vi "SaccadeAnalyser - Main.vi"(8 "error in (no error)":errorcluster, 11 "Data IN":T3={"Impulse Positions"=[{"Start"=5471, "End"=5813, "Impulse Plane"=enum."Yaw", "Impulse Direction +ve?"=FALSE, "Time offset"=0, "Amplitude offset"=0.0}, {"Start"=6974, "End"=7325, "Impulse Plane"=enum."Yaw", "Impulse Direction +ve?"=TRUE, "Time offset"=0, "Amplitude offset"=0.0}, {"Start"=7641, "End"=7980, "Impulse Plane"=enum."Yaw", "Impulse Direction +ve?"=FALSE, "Time offset"=0, "Amplitude offset"=0.0}, {"Start"=9060, "End"=9400, "Impulse Plane"=enum."Yaw", "Impulse Direction +ve?"=FALSE, "Time offset"=0, "Amplitude offset"=0.0}, {"Start"=9938, "End"=10282, "Impulse Plane"=enum."Yaw", "Impulse Direction +ve?"=FALSE, "Time offset"=0, "Amplitude offset"=0.0}, {"Start"=10800, "End"=11142, "Impulse Plane"=enum."Yaw", "Impulse Direction +ve?"=FALSE, "Time offset"=0, "Amplitude offset"=0.0}, {"Start"=11602, "End"=11942, "Impulse Plane"=enum."Yaw", "Impulse Direction +ve?"=TRUE, "Time offset"=0, "Amplitude offset"=0.0}, {"Start"=12449, "End"=12790, "Impulse Plane"=enum."Yaw", "Impulse Direction +ve?"=TRUE, "Time offset"=0, "Amplitude offset"=0.0}, {"Start"=13310, "End"=13653, "Impulse Plane"=enum."Yaw", "Impulse Direction +ve?"=TRUE, "Time offset"=0, "Amplitude offset"=0.0}, {"Start"=14191, "End"=14535, "Impulse Plane"=enum."Yaw", "Impulse Direction +ve?"=TRUE, "Time offset"=0, "Amplitude offset"=0.0}, {"Start"=15040, "End"=15380, "Impulse Plane"=enum."Yaw", "Impulse Direction +ve?"=FALSE, "Time offset"=0, "Amplitude offset"=0.0}, {"Start"=16780, "End"=17124, "Impulse Plane"=enum."Yaw", "Impulse Direction +ve?"=TRUE, "Time offset"=0, "Amplitude offset"=0.0}, {"Start"=17572, "End"=17913, "Impulse Plane"=enum."Yaw", "Impulse Direction +ve?"=FALSE, "Time offset"=0, "Amplitude offset"=0.0}, {"Start"=18369, "End"=18713, "Impulse Plane"=enum."Yaw", "Impulse Direction +ve?"=FALSE, "Time offset"=0, "Amplitude offset"=0.0}, {"Start"=19174, "End"=19519, "Impulse Plane"=enum."Yaw", "Impulse Direction +ve?"=FALSE, "Time offset"=0, "Amplitude offset"=0.0}, {"Start"=19928, "End"=20270, "Impulse Plane"=enum."Yaw", "Impulse Direction +ve?"=TRUE, "Time offset"=0, "Amplitude offset"=0.0}, {"Start"=20762, "End"=21121, "Impulse Plane"=enum."Yaw", "Impulse Direction +ve?"=FALSE, "Time offset"=0, "Amplitude offset"=0.0}, {"Start"=21554, "End"=21888, "Impulse Plane"=enum."Yaw", "Impulse Direction +ve?"=FALSE, "Time offset"=0, "Amplitude offset"=0.0}, {"Start"=22293, "End"=22639, "Impulse Plane"=enum."Yaw", "Impulse Direction +ve?"=TRUE, "Time offset"=0, "Amplitude offset"=0.0}, {"Start"=23109, "End"=23464, "Impulse Plane"=enum."Yaw", "Impulse Direction +ve?"=TRUE, "Time offset"=0, "Amplitude offset"=0.0}, {"Start"=23868, "End"=24215, "Impulse Plane"=enum."Yaw", "Impulse Direction +ve?"=TRUE, "Time offset"=0, "Amplitude offset"=0.0}, {"Start"=24643, "End"=24992, "Impulse Plane"=enum."Yaw", "Impulse Direction +ve?"=FALSE, "Time offset"=0, "Amplitude offset"=0.0}, {"Start"=25685, "End"=26023, "Impulse Plane"=enum."Yaw", "Impulse Direction +ve?"=FALSE, "Time offset"=0, "Amplitude offset"=0.0}, {"Start"=26431, "End"=26768, "Impulse Plane"=enum."Yaw", "Impulse Direction +ve?"=FALSE, "Time offset"=0, "Amplitude offset"=0.0}, {"Start"=27251, "End"=27595, "Impulse Plane"=enum."Yaw", "Impulse Direction +ve?"=FALSE, "Time offset"=0, "Amplitude offset"=0.0}, {"Start"=28832, "End"=29180, "Impulse Plane"=enum."Yaw", "Impulse Direction +ve?"=TRUE, "Time offset"=0, "Amplitude offset"=0.0}, {"Start"=31028, "End"=31383, "Impulse Plane"=enum."LARP", "Impulse Direction +ve?"=FALSE, "Time offset"=0, "Amplitude offset"=0.0}, {"Start"=32603, "End"=32936, "Impulse Plane"=enum."LARP", "Impulse Direction +ve?"=TRUE, "Time offset"=0, "Amplitude offset"=0.0}, {"Start"=33445, "End"=33779, "Impulse Plane"=enum."LARP", "Impulse Direction +ve?"=TRUE, "Time offset"=0, "Amplitude offset"=0.0}, {"Start"=34276, "End"=34629, "Impulse Plane"=enum."LARP", "Impulse Direction +ve?"=FALSE, "Time offset"=0, "Amplitude offset"=0.0}, {"Start"=35114, "End"=35460, "Impulse Plane"=enum."LARP", "Impulse Direction +ve?"=FALSE, "Time offset"=0, "Amplitude offset"=0.0}, {"Start"=35981, "End"=36324, "Impulse Plane"=enum."LARP", "Impulse Direction +ve?"=TRUE, "Time offset"=0, "Amplitude offset"=0.0}, {"Start"=36920, "End"=37249, "Impulse Plane"=enum."LARP", "Impulse Direction +ve?"=TRUE, "Time offset"=0, "Amplitude offset"=0.0}, {"Start"=37988, "End"=38322, "Impulse Plane"=enum."LARP", "Impulse Direction +ve?"=TRUE, "Time offset"=0, "Amplitude offset"=0.0}, {"Start"=38964, "End"=39324, "Impulse Plane"=enum."LARP", "Impulse Direction +ve?"=FALSE, "Time offset"=0, "Amplitude offset"=0.0}, {"Start"=39948, "End"=40284, "Impulse Plane"=enum."LARP", "Impulse Direction +ve?"=TRUE, "Time offset"=0, "Amplitude offset"=0.0}, {"Start"=40958, "End"=41293, "Impulse Plane"=enum."LARP", "Impulse Direction +ve?"=TRUE, "Time offset"=0, "Amplitude offset"=0.0}, {"Start"=41899, "End"=42229, "Impulse Plane"=enum."LARP", "Impulse Direction +ve?"=TRUE, "Time offset"=0, "Amplitude offset"=0.0}, {"Start"=42801, "End"=43154, "Impulse Plane"=enum."LARP", "Impulse Direction +ve?"=FALSE, "Time offset"=0, "Amplitude offset"=0.0}, {"Start"=43641, "End"=43980, "Impulse Plane"=enum."LARP", "Impulse Direction +ve?"=TRUE, "Time offset"=0, "Amplitude offset"=0.0}, {"Start"=44466, "End"=44821, "Impulse Plane"=enum."LARP", "Impulse Direction +ve?"=FALSE, "Time offset"=0, "Amplitude offset"=0.0}, {"Start"=45388, "End"=45722, "Impulse Plane"=enum."LARP", "Impulse Direction +ve?"=TRUE, "Time offset"=0, "Amplitude offset"=0.0}, {"Start"=46149, "End"=46510, "Impulse Plane"=enum."LARP", "Impulse Direction +ve?"=FALSE, "Time offset"=0, "Amplitude offset"=0.0}, {"Start"=47874, "End"=48206, "Impulse Plane"=enum."LARP", "Impulse Direction +ve?"=TRUE, "Time offset"=0, "Amplitude offset"=0.0}, {"Start"=50143, "End"=50479, "Impulse Plane"=enum."RALP", "Impulse Direction +ve?"=TRUE, "Time offset"=0, "Amplitude offset"=0.0}, {"Start"=50976, "End"=51310, "Impulse Plane"=enum."RALP", "Impulse Direction +ve?"=FALSE, "Time offset"=0, "Amplitude offset"=0.0}, {"Start"=51892, "End"=52226, "Impulse Plane"=enum."RALP", "Impulse Direction +ve?"=FALSE, "Time offset"=0, "Amplitude offset"=0.0}, {"Start"=52839, "End"=53171, "Impulse Plane"=enum."RALP", "Impulse Direction +ve?"=FALSE, "Time offset"=0, "Amplitude offset"=0.0}, {"Start"=53676, "End"=54012, "Impulse Plane"=enum."RALP", "Impulse Direction +ve?"=TRUE, "Time offset"=0, "Amplitude offset"=0.0}, {"Start"=54530, "End"=54877, "Impulse Plane"=enum."RALP", "Impulse Direction +ve?"=FALSE, "Time offset"=0, "Amplitude offset"=0.0}, {"Start"=55371, "End"=55711, "Impulse Plane"=enum."RALP", "Impulse Direction +ve?"=TRUE, "Time offset"=0, "Amplitude offset"=0.0}, {"Start"=56153, "End"=56482, "Impulse Plane"=enum."RALP", "Impulse Direction +ve?"=FALSE, "Time offset"=0, "Amplitude offset"=0.0}, {"Start"=57053, "End"=57390, "Impulse Plane"=enum."RALP", "Impulse Direction +ve?"=FALSE, "Time offset"=0, "Amplitude offset"=0.0}, {"Start"=57954, "End"=58292, "Impulse Plane"=enum."RALP", "Impulse Direction +ve?"=FALSE, "Time offset"=0, "Amplitude offset"=0.0}, {"Start"=58794, "End"=59130, "Impulse Plane"=enum."RALP", "Impulse Direction +ve?"=TRUE, "Time offset"=0, "Amplitude offset"=0.0}, {"Start"=59587, "End"=59931, "Impulse Plane"=enum."RALP", "Impulse Direction +ve?"=TRUE, "Time offset"=0, "Amplitude offset"=0.0}, {"Start"=60399, "End"=60744, "Impulse Plane"=enum."RALP", "Impulse Direction +ve?"=FALSE, "Time offset"=0, "Amplitude offset"=0.0}, {"Start"=61218, "End"=61559, "Impulse Plane"=enum."RALP", "Impulse Direction +ve?"=FALSE, "Time offset"=0, "Amplitude offset"=0.0}, {"Start"=62100, "End"=62442, "Impulse Plane"=enum."RALP", "Impulse Direction +ve?"=FALSE, "Time offset"=0, "Amplitude offset"=0.0}, {"Start"=62989, "End"=63322, "Impulse Plane"=enum."RALP", "Impulse Direction +ve?"=FALSE, "Time offset"=0, "Amplitude offset"=0.0}, {"Start"=63787, "End"=64136, "Impulse Plane"=enum."RALP", "Impulse Direction +ve?"=TRUE, "Time offset"=0, "Amplitude offset"=0.0}, {"Start"=64603, "End"=64953, "Impulse Plane"=enum."RALP", "Impulse Direction +ve?"=FALSE, "Time offset"=0, "Amplitude offset"=0.0}, {"Start"=65462, "End"=65795, "Impulse Plane"=enum."RALP", "Impulse Direction +ve?"=FALSE, "Time offset"=0, "Amplitude offset"=0.0}, {"Start"=66308, "End"=66645, "Impulse Plane"=enum."RALP", "Impulse Direction +ve?"=FALSE, "Time offset"=0, "Amplitude offset"=0.0}, {"Start"=67052, "End"=67402, "Impulse Plane"=enum."RALP", "Impulse Direction +ve?"=TRUE, "Time offset"=0, "Amplitude offset"=0.0}], "No. Imp"=15, "Parameter Time Series"=[{"time offset"=0.0, "Offset"=0.0, "Gain"=1.0, "inverse"=FALSE, "filter data"=FALSE, "dots"=FALSE, "interpolate"=FALSE, "List 1"=5, "Color Box"=6618880, "Boolean"=TRUE}, {"time offset"=0.0, "Offset"=0.0, "Gain"=1.0, "inverse"=FALSE, "filter data"=FALSE, "dots"=FALSE, "interpolate"=FALSE, "List 1"=6, "Color Box"=6618880, "Boolean"=FALSE}, {"time offset"=0.0, "Offset"=0.0, "Gain"=1.0, "inverse"=FALSE, "filter data"=FALSE, "dots"=FALSE, "interpolate"=FALSE, "List 1"=7, "Color Box"=6618880, "Boolean"=FALSE}, {"time offset"=0.0, "Offset"=0.0, "Gain"=1.0, "inverse"=FALSE, "filter data"=FALSE, "dots"=FALSE, "interpolate"=FALSE, "List 1"=13, "Color Box"=16777224, "Boolean"=TRUE}, {"time offset"=0.0, "Offset"=0.0, "Gain"=1.0, "inverse"=FALSE, "filter data"=FALSE, "dots"=FALSE, "interpolate"=FALSE, "List 1"=14, "Color Box"=16777224, "Boolean"=FALSE}, {"time offset"=0.0, "Offset"=0.0, "Gain"=1.0, "inverse"=FALSE, "filter data"=FALSE, "dots"=FALSE, "interpolate"=FALSE, "List 1"=15, "Color Box"=16777224, "Boolean"=FALSE}], "Parameter Impuls Series"=[{"Color"=6618880, "Visible"=TRUE, "Channel"=1, "Invert"=FALSE, "Desaccade"=FALSE, "Offset"=0.0, "Gain"=1.0}, {"Color"=6618880, "Visible"=FALSE, "Channel"=6, "Invert"=FALSE, "Desaccade"=FALSE, "Offset"=0.0, "Gain"=1.0}, {"Color"=6618880, "Visible"=FALSE, "Channel"=7, "Invert"=FALSE, "Desaccade"=FALSE, "Offset"=0.0, "Gain"=1.0}, {"Color"=16777224, "Visible"=TRUE, "Channel"=13, "Invert"=FALSE, "Desaccade"=FALSE, "Offset"=0.0, "Gain"=1.0}, {"Color"=16777224, "Visible"=FALSE, "Channel"=14, "Invert"=FALSE, "Desaccade"=FALSE, "Offset"=0.0, "Gain"=1.0}, {"Color"=16777224, "Visible"=FALSE, "Channel"=15, "Invert"=FALSE, "Desaccade"=FALSE, "Offset"=0.0, "Gain"=1.0}], "Experiment Parameters"={"Freq"=0.0, "Vel"=0, "Acc"=0, "Stimulus"="Head Impulse"}, "Autosort File"=refnum, "Data File"={"Data Channels"=array34x71049[2415666 elements], "Sample Rate"=500, "Channel List"=["Hz Position-in-Head", "Hz Velocity-in-Head", "Hy Position-in-Head", "Hy Velocity-in-Head", "Hx Position-in-Head", "Hx Velocity-in-Head", "Hl Velocity-in-Head", "Hr Velocity-in-Head", "Lx Position-in-Head", "Ly Position-in-Head", "Lz Position-in-Head", "Lx Velocity-in-Head", "Ly Velocity-in-Head", "Lz Velocity-in-Head", "Ll Velocity-in-Head", "Lr Velocity-in-Head", "Rx Position-in-Head", "Ry Position-in-Head", "Rz Position-in-Head", "Rx Velocity-in-Head", "Ry Velocity-in-Head", "Rz Velocity-in-Head", "Rl Velocity-in-Head", "Rr Velocity-in-Head", "Target on/off", "aux input 1", "aux input 2", " ", "", "", "", "Target Hor", "Target Ver", ""]}, "Experiment data path"=path "C:/Users/w.figtree/Desktop/Coils Data/3", "Image data path"=path "/Macintosh HD/Users/patrick/Studium/Diploma Thesis/Data Analysis", "LVS data path"=path "/Macintosh HD/Users/patrick/Studium/Diploma Thesis/Data Analysis", "Raw copy path"=path "/Macintosh HD/Users/patrick/Studium/Diploma Thesis/Data Analysis", "filename"="passive_lvs.lvs", "desaccading parameters"={"Tolerance"=3, "Acc Range"=7000.0, "Sample Rate"=500, "Impulse Plane 2"=enum."Yaw", "Impulse dir"=FALSE}, "Experiment Parameters 2"={"Subject"="SE Trial Short Term", "Strain"="", "Rotation plane"="", "Experimenter"=" ", "Trial"=0.0, "Time"=0.0}, "Excel"={"Excel._Application"=refnum, "Use Excel"=TRUE, "Worksheet SINE"=refnum, "Row SINE"=0, "Worksheet TRANS"=refnum, "Row TRANS"=0}, "Session Config File"=refnum, "Autosort Parameter Set"=4, "EMA Version"="EMA 2016a", "desacc "={"Threshold 1 [Acc]"=7000.0, "Threshold 2 [% of TH1]"=60, "tolerance"=3, "Search WD "=0.1, " always use TH2"=FALSE, "Range"=3.0, "Max time"=120.0, "Min time"=20.0, "Velocity Threshold"=150}, "Cycle Nr for Saccades"={"POS"=0, "NEG"=0}, "calibration name"="u_calibration_1_p00001s001_calib.mat", "Excel"=refnum} {"Parameter Time Series"."time offset" format="%.3f"; "Parameter Time Series"."Gain" format="%.1f"; "Parameter Time Series"."Offset" format="%.1f"; "Parameter Time Series"."List 1" items=["Motor-Pos", "Motor-Vel", "Lx Position-in-Head", "Ly Position-in-Head", "Lz Position-in-Head", "Lx Velocity-in-Head", "Ly Velocity-in-Head", "Lz Velocity-in-Head", "Ll Velocity-in-Head", "Lr Velocity-in-Head", "Lx Accel-in-Head", "Ly Accel-in-Head", "Lz Accel-in-Head", "Rx Position-in-Head", "Ry Position-in-Head", "Rz Position-in-Head", "Rx Velocity-in-Head", "Ry Velocity-in-Head", "Rz Velocity-in-Head", "Rl Velocity-in-Head", "Rr Velocity-in-Head", "Rx Accel-in-Head", "Ry Accel-in-Head", "Rz Accel-in-Head", "Global Trigger", "", "", ""]; "Parameter Impuls Series"."Gain" format="%.1f"; "Parameter Impuls Series"."Offset" format="%.1f"}) -> (0 "error out":errorcluster, 3 "Data OUT":T3={"Impulse Positions"=[{"Start"=5471, "End"=5813, "Impulse Plane"=enum."Yaw", "Impulse Direction +ve?"=FALSE, "Time offset"=0, "Amplitude offset"=0.0}, {"Start"=6974, "End"=7325, "Impulse Plane"=enum."Yaw", "Impulse Direction +ve?"=TRUE, "Time offset"=0, "Amplitude offset"=0.0}, {"Start"=7641, "End"=7980, "Impulse Plane"=enum."Yaw", "Impulse Direction +ve?"=FALSE, "Time offset"=0, "Amplitude offset"=0.0}, {"Start"=9060, "End"=9400, "Impulse Plane"=enum."Yaw", "Impulse Direction +ve?"=FALSE, "Time offset"=0, "Amplitude offset"=0.0}, {"Start"=9938, "End"=10282, "Impulse Plane"=enum."Yaw", "Impulse Direction +ve?"=FALSE, "Time offset"=0, "Amplitude offset"=0.0}, {"Start"=10800, "End"=11142, "Impulse Plane"=enum."Yaw", "Impulse Direction +ve?"=FALSE, "Time offset"=0, "Amplitude offset"=0.0}, {"Start"=11602, "End"=11942, "Impulse Plane"=enum."Yaw", "Impulse Direction +ve?"=TRUE, "Time offset"=0, "Amplitude offset"=0.0}, {"Start"=12449, "End"=12790, "Impulse Plane"=enum."Yaw", "Impulse Direction +ve?"=TRUE, "Time offset"=0, "Amplitude offset"=0.0}, {"Start"=13310, "End"=13653, "Impulse Plane"=enum."Yaw", "Impulse Direction +ve?"=TRUE, "Time offset"=0, "Amplitude offset"=0.0}, {"Start"=14191, "End"=14535, "Impulse Plane"=enum."Yaw", "Impulse Direction +ve?"=TRUE, "Time offset"=0, "Amplitude offset"=0.0}, {"Start"=15040, "End"=15380, "Impulse Plane"=enum."Yaw", "Impulse Direction +ve?"=FALSE, "Time offset"=0, "Amplitude offset"=0.0}, {"Start"=16780, "End"=17124, "Impulse Plane"=enum."Yaw", "Impulse Direction +ve?"=TRUE, "Time offset"=0, "Amplitude offset"=0.0}, {"Start"=17572, "End"=17913, "Impulse Plane"=enum."Yaw", "Impulse Direction +ve?"=FALSE, "Time offset"=0, "Amplitude offset"=0.0}, {"Start"=18369, "End"=18713, "Impulse Plane"=enum."Yaw", "Impulse Direction +ve?"=FALSE, "Time offset"=0, "Amplitude offset"=0.0}, {"Start"=19174, "End"=19519, "Impulse Plane"=enum."Yaw", "Impulse Direction +ve?"=FALSE, "Time offset"=0, "Amplitude offset"=0.0}, {"Start"=19928, "End"=20270, "Impulse Plane"=enum."Yaw", "Impulse Direction +ve?"=TRUE, "Time offset"=0, "Amplitude offset"=0.0}, {"Start"=20762, "End"=21121, "Impulse Plane"=enum."Yaw", "Impulse Direction +ve?"=FALSE, "Time offset"=0, "Amplitude offset"=0.0}, {"Start"=21554, "End"=21888, "Impulse Plane"=enum."Yaw", "Impulse Direction +ve?"=FALSE, "Time offset"=0, "Amplitude offset"=0.0}, {"Start"=22293, "End"=22639, "Impulse Plane"=enum."Yaw", "Impulse Direction +ve?"=TRUE, "Time offset"=0, "Amplitude offset"=0.0}, {"Start"=23109, "End"=23464, "Impulse Plane"=enum."Yaw", "Impulse Direction +ve?"=TRUE, "Time offset"=0, "Amplitude offset"=0.0}, {"Start"=23868, "End"=24215, "Impulse Plane"=enum."Yaw", "Impulse Direction +ve?"=TRUE, "Time offset"=0, "Amplitude offset"=0.0}, {"Start"=24643, "End"=24992, "Impulse Plane"=enum."Yaw", "Impulse Direction +ve?"=FALSE, "Time offset"=0, "Amplitude offset"=0.0}, {"Start"=25685, "End"=26023, "Impulse Plane"=enum."Yaw", "Impulse Direction +ve?"=FALSE, "Time offset"=0, "Amplitude offset"=0.0}, {"Start"=26431, "End"=26768, "Impulse Plane"=enum."Yaw", "Impulse Direction +ve?"=FALSE, "Time offset"=0, "Amplitude offset"=0.0}, {"Start"=27251, "End"=27595, "Impulse Plane"=enum."Yaw", "Impulse Direction +ve?"=FALSE, "Time offset"=0, "Amplitude offset"=0.0}, {"Start"=28832, "End"=29180, "Impulse Plane"=enum."Yaw", "Impulse Direction +ve?"=TRUE, "Time offset"=0, "Amplitude offset"=0.0}, {"Start"=31028, "End"=31383, "Impulse Plane"=enum."LARP", "Impulse Direction +ve?"=FALSE, "Time offset"=0, "Amplitude offset"=0.0}, {"Start"=32603, "End"=32936, "Impulse Plane"=enum."LARP", "Impulse Direction +ve?"=TRUE, "Time offset"=0, "Amplitude offset"=0.0}, {"Start"=33445, "End"=33779, "Impulse Plane"=enum."LARP", "Impulse Direction +ve?"=TRUE, "Time offset"=0, "Amplitude offset"=0.0}, {"Start"=34276, "End"=34629, "Impulse Plane"=enum."LARP", "Impulse Direction +ve?"=FALSE, "Time offset"=0, "Amplitude offset"=0.0}, {"Start"=35114, "End"=35460, "Impulse Plane"=enum."LARP", "Impulse Direction +ve?"=FALSE, "Time offset"=0, "Amplitude offset"=0.0}, {"Start"=35981, "End"=36324, "Impulse Plane"=enum."LARP", "Impulse Direction +ve?"=TRUE, "Time offset"=0, "Amplitude offset"=0.0}, {"Start"=36920, "End"=37249, "Impulse Plane"=enum."LARP", "Impulse Direction +ve?"=TRUE, "Time offset"=0, "Amplitude offset"=0.0}, {"Start"=37988, "End"=38322, "Impulse Plane"=enum."LARP", "Impulse Direction +ve?"=TRUE, "Time offset"=0, "Amplitude offset"=0.0}, {"Start"=38964, "End"=39324, "Impulse Plane"=enum."LARP", "Impulse Direction +ve?"=FALSE, "Time offset"=0, "Amplitude offset"=0.0}, {"Start"=39948, "End"=40284, "Impulse Plane"=enum."LARP", "Impulse Direction +ve?"=TRUE, "Time offset"=0, "Amplitude offset"=0.0}, {"Start"=40958, "End"=41293, "Impulse Plane"=enum."LARP", "Impulse Direction +ve?"=TRUE, "Time offset"=0, "Amplitude offset"=0.0}, {"Start"=41899, "End"=42229, "Impulse Plane"=enum."LARP", "Impulse Direction +ve?"=TRUE, "Time offset"=0, "Amplitude offset"=0.0}, {"Start"=42801, "End"=43154, "Impulse Plane"=enum."LARP", "Impulse Direction +ve?"=FALSE, "Time offset"=0, "Amplitude offset"=0.0}, {"Start"=43641, "End"=43980, "Impulse Plane"=enum."LARP", "Impulse Direction +ve?"=TRUE, "Time offset"=0, "Amplitude offset"=0.0}, {"Start"=44466, "End"=44821, "Impulse Plane"=enum."LARP", "Impulse Direction +ve?"=FALSE, "Time offset"=0, "Amplitude offset"=0.0}, {"Start"=45388, "End"=45722, "Impulse Plane"=enum."LARP", "Impulse Direction +ve?"=TRUE, "Time offset"=0, "Amplitude offset"=0.0}, {"Start"=46149, "End"=46510, "Impulse Plane"=enum."LARP", "Impulse Direction +ve?"=FALSE, "Time offset"=0, "Amplitude offset"=0.0}, {"Start"=47874, "End"=48206, "Impulse Plane"=enum."LARP", "Impulse Direction +ve?"=TRUE, "Time offset"=0, "Amplitude offset"=0.0}, {"Start"=50143, "End"=50479, "Impulse Plane"=enum."RALP", "Impulse Direction +ve?"=TRUE, "Time offset"=0, "Amplitude offset"=0.0}, {"Start"=50976, "End"=51310, "Impulse Plane"=enum."RALP", "Impulse Direction +ve?"=FALSE, "Time offset"=0, "Amplitude offset"=0.0}, {"Start"=51892, "End"=52226, "Impulse Plane"=enum."RALP", "Impulse Direction +ve?"=FALSE, "Time offset"=0, "Amplitude offset"=0.0}, {"Start"=52839, "End"=53171, "Impulse Plane"=enum."RALP", "Impulse Direction +ve?"=FALSE, "Time offset"=0, "Amplitude offset"=0.0}, {"Start"=53676, "End"=54012, "Impulse Plane"=enum."RALP", "Impulse Direction +ve?"=TRUE, "Time offset"=0, "Amplitude offset"=0.0}, {"Start"=54530, "End"=54877, "Impulse Plane"=enum."RALP", "Impulse Direction +ve?"=FALSE, "Time offset"=0, "Amplitude offset"=0.0}, {"Start"=55371, "End"=55711, "Impulse Plane"=enum."RALP", "Impulse Direction +ve?"=TRUE, "Time offset"=0, "Amplitude offset"=0.0}, {"Start" (continued)
69.17902917715358, 60.07870769971235, 48.3314198066639, 35.33337743696967, 22.457297716500758, 10.830764991263301, 1.2205986166028433, -6.0146150669211735, -10.892007595538576, -13.694807591178186, -14.851804332650717]}, {[528.0, 530.0, 532.0, 534.0, 536.0, 538.0, 540.0, 542.0, 544.0, 546.0, 548.0, 550.0, 552.0, 554.0, 556.0, 558.0, 560.0, 562.0, 564.0, 566.0000000000001, 568.0000000000001, 570.0000000000001, 572.0000000000001, 574.0000000000001, 576.0000000000001], [-9.527579454864409, -10.577125665129762, -11.131145103375022, -10.584223908245097, -8.348654243177833, -4.004783979283369, 2.5647973786029565, 11.078531818240757, 20.82241073585996, 30.726895783053166, 39.52405801175928, 45.95532417764138, 49.01661960104225, 48.16011299362397, 43.404321671726706, 35.33378791984829, 25.00271709876472, 13.751187200019555, 2.9552038725955043, -6.2063612167617315, -12.921399963820624, -16.839745644954295, -18.071940127929174, -17.104117050659703, -14.654065025286862]}, {[582.0, 584.0, 586.0, 588.0, 590.0, 592.0, 594.0, 596.0, 598.0, 600.0, 602.0, 604.0, 606.0, 608.0, 610.0, 612.0, 614.0, 616.0, 618.0, 620.0, 622.0, 624.0, 626.0, 628.0, 630.0, 632.0, 634.0], [-1.6706932697042873, -3.3455075811287243, -4.473678994481653, -4.396585575335241, -2.4684369191577247, 1.8007580481050427, 8.594949141623625, 17.683034583489096, 28.386913259392607, 39.64175106168615, 50.1408646696851, 58.542587224043245, 63.692457661993835, 64.82578843596133, 61.715514730847474, 54.70461631035364, 44.63458910283943, 32.701219003695016, 20.241708562239864, 8.517446480794685, -1.459609986588287, -9.042719586196379, -13.99397311102634, -16.457101162835592, -16.860363274420028, -15.79407496046417, -13.893778016469078]}, {[474.00000000000006, 476.00000000000006, 478.00000000000006, 480.00000000000006, 482.00000000000006, 484.00000000000006, 486.00000000000006, 488.00000000000006, 490.00000000000006, 492.00000000000006, 494.00000000000006, 496.00000000000006, 498.00000000000006, 500.0, 502.0, 504.0, 506.0, 508.0, 510.0, 512.0, 514.0, 516.0, 518.0, 520.0, 522.0, 524.0, 526.0], [-5.437581721706813, -7.532853000022355, -9.084142746911153, -9.250990048241723, -7.178612795093302, -2.1928649146719312, 6.0140070464960305, 17.233642801887164, 30.675418822257488, 45.01795262576213, 58.59539464359083, 69.67881969840226, 76.76808432526585, 78.8729582975258, 75.70844363988871, 67.73827863726395, 56.07362169336059, 42.251256479738785, 27.958663515334496, 14.743425419148696, 3.764146667680771, -4.34286902425044, -9.463854697830513, -11.922815948161967, -12.338815179197, -11.433286382606058, -9.865105428418754]}, {[564.0, 566.0000000000001, 568.0000000000001, 570.0000000000001, 572.0000000000001, 574.0000000000001, 576.0000000000001, 578.0000000000001, 580.0000000000001, 582.0000000000001, 584.0000000000001, 586.0000000000001, 588.0000000000001, 590.0000000000001, 592.0000000000001, 594.0000000000001, 596.0000000000001, 598.0000000000001, 600.0000000000001, 602.0000000000001, 604.0000000000001, 606.0000000000001, 608.0000000000001, 610.0000000000001, 612.0000000000001, 614.0000000000001, 616.0000000000001], [-9.080046765081676, -10.678128490411645, -11.6707704891704, -11.469856027373027, -9.5158355327974, -5.413075001297588, 0.9434399127670785, 9.27089343229068, 18.885806355145963, 28.78298155221996, 37.772096486182164, 44.65829905955033, 48.46266031046852, 48.61309811323283, 45.03993832436139, 38.180486368387854, 28.912453408573064, 18.402759339239452, 7.886075499642308, -1.5232402772824392, -8.985318767842745, -14.04591575558494, -16.647938966841256, -17.078934812254147, -15.873611988630202, -13.67825841551836, -11.126693516226487]}, {[518.0, 520.0, 522.0, 524.0, 526.0, 528.0, 530.0, 532.0, 534.0, 536.0, 538.0, 540.0, 542.0, 544.0, 546.0, 548.0, 550.0, 552.0, 554.0, 556.0, 558.0, 560.0, 562.0, 564.0, 566.0000000000001, 568.0000000000001, 570.0000000000001], [-11.4476193776905, -13.068851678881895, -13.862730914838576, -12.99963998702583, -9.694639981902103, -3.402083180014002, 6.032556885524558, 18.251678113366445, 32.3514578152284, 46.96196273804698, 60.41458212174757, 71.01485846520777, 77.33772940656948, 78.468047531521, 74.18538908447246, 65.01631412660365, 52.128564083566516, 37.14123702954777, 21.855399138477154, 7.934316510732438, -3.3578249787371295, -11.309186108976784, -15.805578117508423, -17.26506975033719, -16.46631522978143, -14.335344694369246, -11.750138041033814]}, {[498.0, 500.0, 502.0, 504.0, 506.0, 508.0, 510.0, 512.0, 514.0, 516.0, 518.0, 520.0, 522.0, 524.0, 526.0, 528.0, 530.0, 532.0, 534.0, 536.0, 538.0, 540.0, 542.0, 544.0, 546.0, 548.0, 550.0], [-0.012091313230288447, -1.7421638804518995, -3.0389623640143157, -3.245396673757427, -1.6948480326152768, 2.1384328191819306, 8.469521915823595, 17.087054841087145, 27.315418397717107, 38.05757322742741, 47.94620610349132, 55.57948276025742, 59.777197966332054, 59.80311209652382, 55.50908234625477, 47.38023657915541, 36.450375305358186, 24.101455072542254, 11.809603266892601, 0.8926245665691606, -7.699270570892281, -13.502462377823814, -16.541721280039642, -17.24392262332151, -16.284433481949875, -14.412508844326226, -12.2971280291156]}, {[554.0, 556.0, 558.0, 560.0, 562.0, 564.0, 566.0000000000001, 568.0000000000001, 570.0000000000001, 572.0000000000001, 574.0000000000001, 576.0000000000001, 578.0000000000001, 580.0000000000001, 582.0000000000001, 584.0000000000001, 586.0000000000001, 588.0000000000001, 590.0000000000001, 592.0000000000001, 594.0000000000001, 596.0000000000001, 598.0000000000001, 600.0000000000001, 602.0000000000001, 604.0000000000001, 606.0000000000001], [-4.522231629389672, -6.099356541635326, -7.033837566184765, -6.530522920748879, -3.7817473387038465, 1.850754719532537, 10.642426983685915, 22.365587411552568, 36.23501199222388, 50.94709617216887, 64.84101602206391, 76.17471628829185, 83.41922636843152, 85.51991298092757, 82.09980450239388, 73.53608919952723, 60.89872991717725, 45.758420318077484, 29.907265361805152, 15.058407133564199, 2.5737382904767507, -6.715899336652479, -12.57598159697483, -15.3246447501556, -15.686631915632411, -14.574916517929267, -12.872113276125042]}, {[520.0, 522.0, 524.0, 526.0, 528.0, 530.0, 532.0, 534.0, 536.0, 538.0, 540.0, 542.0, 544.0, 546.0, 548.0, 550.0, 552.0, 554.0, 556.0, 558.0, 560.0, 562.0, 564.0, 566.0000000000001, 568.0000000000001, 570.0000000000001, 572.0000000000001], [-7.500446204332798, -8.149769047301705, -8.599376666418916, -8.441802829436932, -7.230678641797557, -4.591111049576478, -0.3257926505220681, 5.492766404293648, 12.473385539202374, 19.915354566494162, 26.90003759789026, 32.44825466462659, 35.686366632079164, 36.01778064482943, 33.26105823585337, 27.682301361140524, 19.94926639447815, 11.04003883936146, 2.0609526551163264, -5.955707230259444, -12.201977016180082, -16.200494428585834, -17.8432974158248, -17.366919156986576, -15.269937620203358, -12.180213398484451, -8.726924390155432]}, {[552.0, 554.0, 556.0, 558.0, 560.0, 562.0, 564.0, 566.0000000000001, 568.0000000000001, 570.0000000000001, 572.0000000000001, 574.0000000000001, 576.0000000000001, 578.0000000000001, 580.0000000000001, 582.0000000000001, 584.0000000000001, 586.0000000000001, 588.0000000000001, 590.0000000000001, 592.0000000000001, 594.0000000000001, 596.0000000000001, 598.0000000000001, 600.0000000000001, 602.0000000000001, 604.0000000000001], [-7.176035360345667, -7.398600739376963, -7.3767525082011804, -6.7782328355304795, -5.314655641339901, -2.8256467063059447, 0.6726090248953283, 4.98148672460113, 9.750320796626117, 14.530187559033408, 18.84255920678958, 22.26067541171979, 24.468305768199688, 25.29294718130975, 24.725614427990152, 22.9030335665933, 20.082655608922238, 16.606151876437476, 12.82963888753322, 9.079726996951507, 5.622531347536689, 2.6217090367480265, 0.13171202491932155, -1.8838458215461478, -3.5233802618856194, -4.91150074028557, -6.173130009585858]}, {[552.0, 554.0, 556.0, 558.0, 560.0, 562.0, 564.0, 566.0000000000001, 568.0000000000001, 570.0000000000001, 572.0000000000001, 574.0000000000001, 576.0000000000001, 578.0000000000001, 580.0000000000001, 582.0000000000001, 584.0000000000001, 586.0000000000001, 588.0000000000001, 590.0000000000001, 592.0000000000001, 594.0000000000001, 596.0000000000001, 598.0000000000001, 600.0000000000001, 602.0000000000001], [-7.038075410780015, -8.577769843416434, -9.850303709444205, -10.436079719799327, -9.89643731331821, -7.860113468983564, -4.139867507193869, 1.1836393543016275, 7.714366955283603, 14.747407872743832, 21.37706522917261, 26.656315254909103, 29.755925905755753, 30.1306788554151, 27.65294175194612, 22.631211021641793, 15.742249750023644, 7.917552080655157, 0.16434731585808038, -6.624286177975039, -11.814424012090928, -15.105823184589445, -16.53122154971252, -16.40521618929207, -15.215912519074433, -13.498067256588318]}, {[0.0, 2.0, 4.0, 6.0, 8.0, 10.0, 12.0, 14.0, 16.0, 18.000000000000004, 20.0, 22.0, 24.0, 26.000000000000004, 28.0, 30.0, 32.0, 34.0, 36.00000000000001, 38.0, 40.0, 42.0, 44.0, 46.0, 48.0, 50.0, 52.00000000000001, 54.0, 56.0, 58.0, 60.0, 62.0, 64.0, 66.0, 68.0, 70.0, 72.00000000000001, 74.0, 76.0, 78.0, 80.0, 82.0, 84.0, 86.0, 88.0, 90.0, 92.0, 94.0, 96.0, 98.0, 100.0, 102.00000000000001, 104.00000000000001, 106.0, 108.0, 110.0, 112.0, 114.0, 116.0, 118.00000000000001, 120.0, 122.0, 124.0, 126.0, 128.0, 130.0, 132.0, 134.0, 136.0, 138.0, 140.0, 142.00000000000003, 144.00000000000003, 146.0, 148.0, 150.0, 152.0, 154.0, 156.0, 158.0, 160.0, 162.0, 164.0, 166.0, 168.0, 170.0, 172.0, 174.00000000000003, 176.0, 178.0, 180.0, 182.0, 184.0, 186.0, 188.0, 190.0, 192.0, 194.0, 196.0, 198.0, 200.0, 202.0, 204.00000000000003, 206.00000000000003, 208.00000000000003, 210.0, 212.0, 214.0, 216.0, 218.0, 220.0, 222.0, 224.0, 226.0, 228.0, 230.0, 232.0, 234.0, 236.00000000000003, 238.00000000000003, 240.0, 242.0, 244.0, 246.0, 248.0, 250.0, 252.0, 254.0, 256.0, 258.0, 260.0, 262.0, 264.0, 266.0, 268.0, 270.0, 272.0, 274.0, 276.0, 278.0, 280.0, 282.0, 284.00000000000006, 286.00000000000006, 288.00000000000006, 290.0, 292.0, 294.0, 296.0, 298.0, 300.0, 302.0, 304.0, 306.0, 308.0, 310.0, 312.0, 314.0, 316.0, 318.0, 320.0, 322.0, 324.0, 326.0, 328.0, 330.0, 332.0, 334.0, 336.0, 338.0, 340.0, 342.0, 344.0, 346.00000000000006, 348.00000000000006, 350.00000000000006, 352.0, 354.0, 356.0, 358.0, 360.0, 362.0, 364.0, 366.0, 368.0, 370.0, 372.0, 374.0, 376.0, 378.0, 380.0, 382.0, 384.0, 386.0, 388.0, 390.0, 392.0, 394.0, 396.0, 398.0, 400.0, 402.0, 404.0, 406.0, 408.00000000000006, 410.00000000000006, 412.00000000000006, 414.00000000000006, 416.00000000000006, 418.0, 420.0, 422.0, 424.0, 426.0, 428.0, 430.0, 432.0, 434.0, 436.0, 438.0, 440.0, 442.0, 444.0, 446.0, 448.0, 450.0, 452.0, 454.0, 456.0, 458.0, 460.0, 462.0, 464.0, 466.0, 468.0, 470.00000000000006, 472.00000000000006, 474.00000000000006, 476.00000000000006, 478.00000000000006, 480.0, 482.0, 484.0, 486.0, 488.0, 490.0, 492.0, 494.0, 496.0, 498.0, 500.0, 502.0, 504.0, 506.0, 508.0, 510.0, 512.0, 514.0, 516.0, 518.0, 520.0, 522.0, 524.0, 526.0, 528.0, 530.0, 532.0, 534.0, 536.0, 538.0, 540.0, 542.0, 544.0, 546.0, 548.0, 550.0, 552.0, 554.0, 556.0, 558.0, 560.0, 562.0, 564.0, 566.0000000000001, 568.0000000000001, 570.0000000000001, 572.0000000000001, 574.0000000000001, 576.0000000000001, 578.0, 580.0, 582.0, 584.0, 586.0, 588.0, 590.0, 592.0, 594.0, 596.0, 598.0, 600.0, 602.0, 604.0, 606.0, 608.0, 610.0, 612.0, 614.0, 616.0, 618.0, 620.0, 622.0, 624.0, 626.0, 628.0, 630.0, 632.0, 634.0, 636.0, 638.0, 640.0, 642.0, 644.0, 646.0, 648.0, 650.0, 652.0, 654.0, 656.0, 658.0, 660.0, 662.0, 664.0, 666.0, 668.0], [-0.06389984985435682, -0.12570215489812853, -0.18723624777264014, -0.23828621839494524, -0.2694747074102395, -0.27642488116316066, -0.2565836311633518, -0.20727945016965776, -0.1343952403934754, -0.05130262808294894, 0.026136502806187067, 0.09013326590404347, 0.13607030565691858, 0.1528909675810457, 0.13442869149282366, 0.07988100427413869, -0.002401488036655408, -0.1022500676685194, -0.21797896262421368, -0.3388258429025601, -0.44434173621161754, -0.5193440654063686, -0.5441483456323404, -0.49032714150705736, -0.33793533239258977, -0.0807577811775344, 0.2709286369262154, 0.6842131468323549, 1.1059532487254442, 1.4712547669651963, 1.7184375078906475, 1.8037877183406046, 1.7165562417297897, 1.4906890339021412, 1.1962647788928518, 0.9219480164005205, 0.7556012152472324, 0.7566134320243072, 0.9375918220718509, 1.2604732475075489, 1.6373372725704858, 1.9502489127578508, 2.0859920093783213, 1.9667398372264877, 1.571410782977047, 0.9479237512795624, 0.20652338004889703, -0.5061423952844164, -1.036944621211461, -1.2653053318499596, -1.1309933377401444, -0.6366869285332228, 0.15166053693547, 1.1156729380654244, 2.11318603669417, 3.0055200477133646, 3.6859144692725643, 4.094720432450903, 4.215302256662561, 4.0766289401086775, 3.742633925618021, 3.30620501255844, 2.881439696264434, 2.574878674689037, 2.4803761037274317, 2.6706236208689536, 3.18368074995124, 4.007194511359277, 5.0710977588308666, 6.268854508144667, 7.469526323813759, 8.530376261036054, 9.342553263713715, 9.863799207277001, 10.123466542701575, 10.229880290219269, 10.354131182709867, 10.696877627531286, 11.45321245373188, 12.780097146857049, 14.755224840526338, 17.357696457903977, 20.48998681579132, 23.99995799476212, 27.706546163615634, 31.431952854451144, 35.04133998301175, 38.468242825404246, 41.71242171435395, 44.83963375223422, 47.96908344679959, 51.24060422237642, 54.79190574811583, 58.740443124718546, 63.155006680308226, 68.04465837590038, 73.3615702443747, 79.00358082817246, 84.83319830639687, 90.69733687089266, 96.4423992300049, 101.9432307418265, 107.12399871295318, 111.95524640951494, 116.44863508113531, 120.6472053453836, 124.60196091677193, 128.349142018269, 131.89713260435985, 135.21463691584137, 138.22863339329965, 140.84690778164585, 142.9860874893099, 144.58344412978295, 145.60554802558585, 146.06292399523926, 146.0050494698197, 145.49918498468293, 144.61919601487403, 143.4294723740994, 141.9684488682583, 140.25116736087017, 138.28057416903903, 136.05354532550473, 133.57377096057576, 130.8644435484759, 127.96387751830784, 124.91429647774994, 121.74804633491232, 118.48705031725001, 115.12902939470527, 111.63761756623985, 107.9664649494672, 104.08208868515223, 99.97245653901649, 95.64179125464611, 91.12366744477903, 86.48787454792571, 81.81316742172847, 77.17316323413405, 72.6261348434492, 68.19300745085101, 63.864589153901576, 59.612788560229006, 55.389694447532946, 51.14642940264445, 46.84700990973632, 42.46941103237013, 38.014749206524115, 33.516721174253604, 29.028002933027782, 24.607030786188567, 20.326059759819604, 16.26756107893855, 12.503978941178676, 9.094780849860012, 6.086096366431338, 3.49866889030888, 1.3247104029809376, -0.48371886388815666, -2.0177722903845234, -3.393651881805288, -4.733521672382471, -6.143625357696668, -7.698555384136507, -9.425089192371736, -11.291206743853799, -13.206870439337532, -15.03853142345734, -16.649724144701665, -17.932941410231564, -18.814981304641147, -19.281357424128956, -19.393016423724085, -19.26490623139781, -19.03918123787503, -18.857271067575972, -18.83815084441698, -19.048711735356235, -19.481946575012877, -20.070198718358654, -20.70829324652221, -21.278554039911622, -21.67428152886609, -21.82600379548085, -21.732919189201056, -21.45993044115803, -21.109104979904828, -20.78788405459494, -20.581721175833167, -20.54113979532611, -20.660261440958287, -20.86262045188685, -21.02819124115802, -21.03757725352456, -20.797510556960738, -20.26030784475326, -19.439735515361683, -18.408533466274093, -17.27478134191867, -16.154037997324632, -15.148545262331227, -14.31686352558911, -13.66225116467085, -13.15704653269165, -12.75387164805027, -12.392129406286909, -12.024811564114465, -11.63692544379666, -11.241171953338721, -10.863122731837592, -10.52960912628934, -10.258073831383156, -10.04868665772845, -9.879755866486377, -9.715367173222496, -9.52530000995492, -9.286537202165821, -8.984146165670936, -8.630912304170035, -8.267568565427151, -7.9366125762916955, -7.679960446571975, -7.542205570373248, -7.547693321484007, -7.684364581657373, -7.911633348135986, -8.179315069141527, -8.41855546194656, -8.549571489449557, -8.518307893037509, -8.302060451762626, -7.918675856486931, -7.436473975500149, -6.955523665965402, -6.58891068598745, -6.4467335298213095, -6.60563125019346, -7.073137408571714, -7.788658924187796, -8.634927391988677, -9.449305857255634, -10.061179740092758, -10.323049141832405, -10.146512866779464, -9.536370639676214, -8.592198325897762, -7.495574612435697, -6.498709060387066, -5.888672615388614, -5.9297582067843715, -6.801976189574921, -8.523709941509901, -10.902101120878495, -13.515153937729416, -15.705975171447783, -16.647195116153465, -15.47020228179682, -11.434549595782723, -4.102893640842959, 6.514226198648548, 19.860845176201657, 34.84648813171131, 49.95971640001052, 63.47724286885524, 73.74340864036043, 79.44374271664638, 79.83243426595925, 74.86210287260596, 65.19120077463768, 52.06529031428731, 37.08937138080604, 21.955981839601936, 8.17411492228468, -3.1425345306333585, -11.379811752888802, -16.44083754969223, -18.678736575190545, -18.73357784286452, -17.361621097688346, -15.295562056242597, -13.126955560682532, -11.25919027367259, -9.902590375807705, -9.105508127115133, -8.811095023693332, -8.908120326942106, -9.278464792543527, -9.809734471536736, -10.406083214014668, -10.985107186987104, -11.465988096160327, -11.787713363457426, -11.903355748655049, -11.780252379804178, -11.424703283907315, -10.887481362002578, -10.256370045699205, -9.647784475150074, -9.182800422268835, -8.962330485598457, -9.048730538129586, -9.436451299028075, -10.061297123891809, -10.825541930948006, -11.605459832539808, -12.284854198216514, -12.782618524602857, -13.069442822392013, -13.16413538408003, -13.10861000890045, -12.972535989288883, -12.833269358890059, -12.747813838612457, -12.755093207153905, -12.872929958591776, -13.106784357022635, -13.453068220901375, -13.895288578073693, -14.408071067723945, -14.953077011804368, -15.480409837741815, -15.937449333891552, -16.278852147040272, -16.481496955242093, -16.551989944571563, -16.52724570290065, -16.475929940625278, -16.477651696261315, -16.593795926374227, -16.85360692625831, -17.240169169498316, -17.687782930024753, -18.094286230074253]}, {[0.0, 2.0, 4.0, 6.0, 8.0, 10.0, 12.0, 14.0, 16.0, 18.000000000000004, 20.0, 22.0, 24.0, 26.000000000000004, 28.0, 30.0, 32.0, 34.0, 36.00000000000001, 38.0, 40.0, 42.0, 44.0, 46.0, 48.0, 50.0, 52.00000000000001, 54.0, 56.0, 58.0, 60.0, 62.0, 64.0, 66.0, 68.0, 70.0, 72.00000000000001, 74.0, 76.0, 78.0, 80.0, 82.0, 84.0, 86.0, 88.0, 90.0, 92.0, 94.0, 96.0, 98.0, 100.0, 102.00000000000001, 104.00000000000001, 106.0, 108.0, 110.0, 112.0, 114.0, 116.0, 118.00000000000001, 120.0, 122.0, 124.0, 126.0, 128.0, 130.0, 132.0, 134.0, 136.0, 138.0, 140.0, 142.00000000000003, 144.00000000000003, 146.0, 148.0, 150.0, 152.0, 154.0, 156.0, 158.0, 160.0, 162.0, 164.0, 166.0, 168.0, 170.0, 172.0, 174.00000000000003, 176.0, 178.0, 180.0, 182.0, 184.0, 186.0, 188.0, 190.0, 192.0, 194.0, 196.0, 198.0, 200.0, 202.0, 204.00000000000003, 206.00000000000003, 208.00000000000003, 210.0, 212.0, 214.0, 216.0, 218.0, 220.0, 222.0, 224.0, 226.0, 228.0, 230.0, 232.0, 234.0, 236.00000000000003, 238.00000000000003, 240.0, 242.0, 244.0, 246.0, 248.0, 250.0, 252.0, 254.0, 256.0, 258.0, 260.0, 262.0, 264.0, 266.0, 268.0, 270.0, 272.0, 274.0, 276.0, 278.0, 280.0, 282.0, 284.00000000000006, 286.00000000000006, 288.00000000000006, 290.0, 292.0, 294.0, 296.0, 298.0, 300.0, 302.0, 304.0, 306.0, 308.0, 310.0, 312.0, 314.0, 316.0, 318.0, 320.0, 322.0, 324.0, 326.0, 328.0, 330.0, 332.0, 334.0, 336.0, 338.0, 340.0, 342.0, 344.0, 346.00000000000006, 348.00000000000006, 350.00000000000006, 352.0, 354.0, 356.0, 358.0, 360.0, 362.0, 364.0, 366.0, 368.0, 370.0, 372.0, 374.0, 376.0, 378.0, 380.0, 382.0, 384.0, 386.0, 388.0, 390.0, 392.0, 394.0, 396.0, 398.0, 400.0, 402.0, 404.0, 406.0, 408.00000000000006, 410.00000000000006, 412.00000000000006, 414.00000000000006, 416.00000000000006, 418.0, 420.0, 422.0, 424.0, 426.0, 428.0, 430.0, 432.0, 434.0, 436.0, 438.0, 440.0, 442.0, 444.0, 446.0, 448.0, 450.0, 452.0, 454.0, 456.0, 458.0, 460.0, 462.0, 464.0, 466.0, 468.0, 470.00000000000006, 472.00000000000006, 474.00000000000006, 476.00000000000006, 478.00000000000006, 480.0, 482.0, 484.0, 486.0, 488.0, 490.0, 492.0, 494.0, 496.0, 498.0, 500.0, 502.0, 504.0, 506.0, 508.0, 510.0, 512.0, 514.0, 516.0, 518.0, 520.0, 522.0, 524.0, 526.0, 528.0, 530.0, 532.0, 534.0, 536.0, 538.0, 540.0, 542.0, 544.0, 546.0, 548.0, 550.0, 552.0, 554.0, 556.0, 558.0, 560.0, 562.0, 564.0, 566.0000000000001, 568.0000000000001, 570.0000000000001, 572.0000000000001, 574.0000000000001, 576.0000000000001, 578.0, 580.0, 582.0, 584.0, 586.0, 588.0, 590.0, 592.0, 594.0, 596.0, 598.0, 600.0, 602.0, 604.0, 606.0, 608.0, 610.0, 612.0, 614.0, 616.0, 618.0, 620.0, 622.0, 624.0, 626.0, 628.0, 630.0, 632.0, 634.0, 636.0, 638.0, 640.0, 642.0, 644.0, 646.0, 648.0, 650.0, 652.0, 654.0, 656.0, 658.0, 660.0, 662.0, 664.0, 666.0, 668.0], [0.06458253579902262, 0.12641747205971576, 0.19096335123860264, 0.24849305434333147, 0.28941208333642265, 0.30612395877622767, 0.2945778793908431, 0.2551943763644484, 0.19301381301139742, 0.11699128071602338, 0.04131407242294394, -0.021673725233879892, -0.06632776260808448, -0.085636812250792, -0.07255032321771893, -0.027240625772188665, 0.0390880035338963, 0.11599140679800435, 0.19962189958109633, 0.28071156284778276, 0.3482492791213776, 0.395042698770359, 0.41543788269957105, 0.4055567428894218, 0.36392841232424367, 0.292268386076314, 0.19551895451989587, 0.08086094715915948, -0.04413473487649622, -0.17297144427726696, -0.3025629136587362, -0.4327019998116386, -0.5671847713349756, -0.717460675381612, -0.8953987427580978, -1.106882676556208, -1.3505730732150218, -1.611480531748441, -1.8615399945011788, -2.066184442826123, -2.182192350451393, -2.1678327604288015, -2.0018522059252524, -1.6874819642211891, -1.2530648175959103, -0.7557024833465311, -0.2735140217528498, 0.11159456955975333, 0.32760977683311143, 0.3319751965407205, 0.12162500967059575, -0.27699028641311063, -0.812823042304486, -1.4156683204195142, -2.0166355706760797, -2.567666355039921, -3.0450599944718277, -3.4453786697339823, -3.781504678671581, -4.07641693517087, -4.349399200950554, -4.609648620788203, -4.861608090823473, -5.102842009313946, -5.329873101741815, -5.552914105736262, -5.801014197524002, -6.107808785363408, -6.500363165793188, -6.999675543459633, -7.6079152354948185, -8.299807571401473, -9.037100841707609, -9.784155213160194, -10.524344658762917, -11.277319283479436, -12.09891563083352, -13.076645107403394, -14.31423118111405, -15.909622340151365, -17.926626069349506, -20.372518259426286, -23.20580407420573, -26.347272177160587, -29.69203956535824, -33.13237161425805, -36.58608480401271, -40.013720124925996, -43.415281319838705, -46.829130294334874, -50.319147866072186, -53.94954756497235, -57.77693868050195, -61.84172857835172, -66.15181349829044, -70.68529217334041, -75.39886197807456, -80.22823258454807, -85.09733714236886, -89.922208494132, -94.60859709239733, -99.06659692059245, -103.22375564441077, -107.02135515489744, -110.42265342540203, -113.4255565902019, -116.05421028991572, -118.34953000717331, -120.36158391022306, -122.13248587207315, -123.68956120654332, -125.04387224097823, -126.18701773512905, -127.09922730092646, -127.75472551444366, -128.12520338074992, -128.1859611069718, -127.91376739361465, -127.28772278191227, -126.29176964629147, -124.91583175944822, -123.1611682788122, -121.04993539415759, -118.62641955703032, -115.9570712252837, -113.12902865506783, -110.23018801037804, -107.33500899237023, -104.48523326994474, -101.6800200949063, -98.8797761533678, -96.01058717275987, -92.98842888197724, -89.74686603399309, -86.25364267194877, -82.50846062372369, -78.54735629734529, -74.44210465183335, -70.27059597927817, -66.10067903561279, -61.98132638268148, -57.92464738331248, -53.91788344278221, -49.93849268217218, -45.95428000540507, -41.93744315756994, -37.876185639257656, -33.775208904458026, -29.65590766482311, -25.56132016358209, -21.545654917211465, -17.66300783327436, -13.97641969743785, -10.555232115504102, -7.45555642634231, -4.717240056070696, -2.3646785343519396, -0.3952665474185526, 1.2203639445618397, 2.538134086361227, 3.638423733824953, 4.612620109503929, 5.550120450625389, 6.522237324541447, 7.577973193782813, 8.74605304286703, 10.026845244585212, 11.390737332245784, 12.787102982936805, 14.15852184086376, 15.444913118083917, 16.577986162057822, 17.4975614576618, 18.168250607364737, 18.582749849315263, 18.76711507509402, 18.779353850185906, 18.700594031051573, 18.61663579961636, 18.598136911241085, 18.683075132646525, 18.861718793989887, 19.083209738170293, 19.27059616161004, 19.334922254388303, 19.211893861408065, 18.887327733055105, 18.39483030538951, 17.80473048668201, 17.20591120012508, 16.687463091100412, 16.309226322381743, 16.07007003565395, 15.914743701499145, 15.760758253328135, 15.515759704438235, 15.102896899441737, 14.483869657386467, 13.672375110996214, 12.72998910539331, 11.74480398075213, 10.810523896707378, 9.998409499592874, 9.339735666958637, 8.836702787710452, 8.464329476297879, 8.171550015318164, 7.9124641939555325, 7.664417155813025, 7.419883682869085, 7.185287230343198, 6.975823861497373, 6.8009792844750265, 6.657285445607851, 6.526210673902147, 6.382484337564493, 6.206464679790177, 5.984034475602367, 5.715105886024807, 5.429718783929197, 5.175360667867455, 4.9909679654054955, 4.908117666609526, 4.950552938590192, 5.1173621954796715, 5.378037398621763, 5.68325836373498, 5.984064685181609, 6.227715857867647, 6.364996614336652, 6.375248317231956, 6.253810546619962, 6.010614282836809, 5.684245984270282, 5.3240463662679165, 4.9763473255864, 4.689726092977042, 4.505328207122584, 4.4407227823946585, 4.496105054176425, 4.659962689167125, 4.909105727295275, 5.21646051187371, 5.556259855959323, 5.908086656810592, 6.257636232256877, 6.592816759028215, 6.897768966764337, 7.156707887690793, 7.356398968396791, 7.487223791413319, 7.552803873805497, 7.565630736839314, 7.550587337171713, 7.550670481820406, 7.603078351110387, 7.724347076643449, 7.916060376986998, 8.163036969257593, 8.426888738037766, 8.657931819596008, 8.812254157536067, 8.858978302319542, 8.795881494184169, 8.653209593813127, 8.48038036152824, 8.332838306007755, 8.25706218484064, 8.283046995847604, 8.413865618587792, 8.619443359031264, 8.843150232245044, 9.020250836849009, 9.105664553086179, 9.078305910565515, 8.934461606156852, 8.6954816726816, 8.409133294573968, 8.118606658492778, 7.848790449842461, 7.615705054994875, 7.418081518321353, 7.2470679251346475, 7.099962610628195, 6.98425391886346, 6.917478725480834, 6.923743288938286, 7.030416389854556, 7.245273322375143, 7.550829055786391, 7.905773018099132, 8.246054728066046, 8.512379168377542, 8.66071689044085, 8.667436109674401, 8.546508246965704, 8.349500606955534, 8.151300017963642, 8.032491053170112, 8.052474982488377, 8.232894488099502, 8.557924956421227, 8.968366544745622, 9.384455248204098, 9.738444385180362, 9.983461023491895, 10.111221357647029, 10.16181347372123, 10.212856329515638, 10.34981905868743, 10.634342323615877, 11.095085399355508, 11.710152679622624, 12.406149533285669, 13.086692257023383, 13.650826090715972, 14.020496374865836, 14.164195224206608, 14.101424499926651, 13.898137530934143, 13.647721701909296, 13.446275336376383, 13.370982494648157, 13.465009935980895, 13.730071436738852, 14.129316790294677, 14.599133156073869, 15.071287123152112, 15.485597990748863, 15.79619991007555, 15.987504577824506, 16.070150696550606, 16.066608481702342, 16.004980237188775]}, {[0.0, 2.0, 4.0, 6.0, 8.0, 10.0, 12.0, 14.0, 16.0, 18.000000000000004, 20.0, 22.0, 24.0, 26.000000000000004, 28.0, 30.0, 32.0, 34.0, 36.00000000000001, 38.0, 40.0, 42.0, 44.0, 46.0, 48.0, 50.0, 52.00000000000001, 54.0, 56.0, 58.0, 60.0, 62.0, 64.0, 66.0, 68.0, 70.0, 72.00000000000001, 74.0, 76.0, 78.0, 80.0, 82.0, 84.0, 86.0, 88.0, 90.0, 92.0, 94.0, 96.0, 98.0, 100.0, 102.00000000000001, 104.00000000000001, 106.0, 108.0, 110.0, 112.0, 114.0, 116.0, 118.00000000000001, 120.0, 122.0, 124.0, 126.0, 128.0, 130.0, 132.0, 134.0, 136.0, 138.0, 140.0, 142.00000000000003, 144.00000000000003, 146.0, 148.0, 150.0, 152.0, 154.0, 156.0, 158.0, 160.0, 162.0, 164.0, 166.0, 168.0, 170.0, 172.0, 174.00000000000003, 176.0, 178.0, 180.0, 182.0, 184.0, 186.0, 188.0, 190.0, 192.0, 194.0, 196.0, 198.0, 200.0, 202.0, 204.00000000000003, 206.00000000000003, 208.00000000000003, 210.0, 212.0, 214.0, 216.0, 218.0, 220.0, 222.0, 224.0, 226.0, 228.0, 230.0, 232.0, 234.0, 236.00000000000003, 238.00000000000003, 240.0, 242.0, 244.0, 246.0, 248.0, 250.0, 252.0, 254.0, 256.0, 258.0, 260.0, 262.0, 264.0, 266.0, 268.0, 270.0, 272.0, 274.0, 276.0, 278.0, 280.0, 282.0, 284.00000000000006, 286.00000000000006, 288.00000000000006, 290.0, 292.0, 294.0, 296.0, 298.0, 300.0, 302.0, 304.0, 306.0, 308.0, 310.0, 312.0, 314.0, 316.0, 318.0, 320.0, 322.0, 324.0, 326.0, 328.0, 330.0, 332.0, 334.0, 336.0, 338.0, 340.0, 342.0, 344.0, 346.00000000000006, 348.00000000000006, 350.00000000000006, 352.0, 354.0, 356.0, 358.0, 360.0, 362.0, 364.0, 366.0, 368.0, 370.0, 372.0, 374.0, 376.0, 378.0, 380.0, 382.0, 384.0, 386.0, 388.0, 390.0, 392.0, 394.0, 396.0, 398.0, 400.0, 402.0, 404.0, 406.0, 408.00000000000006, 410.00000000000006, 412.00000000000006, 414.00000000000006, 416.00000000000006, 418.0, 420.0, 422.0, 424.0, 426.0, 428.0, 430.0, 432.0, 434.0, 436.0, 438.0, 440.0, 442.0, 444.0, 446.0, 448.0, 450.0, 452.0, 454.0, 456.0, 458.0, 460.0, 462.0, 464.0, 466.0, 468.0, 470.00000000000006, 472.00000000000006, 474.00000000000006, 476.00000000000006, 478.00000000000006, 480.0, 482.0, 484.0, 486.0, 488.0, 490.0, 492.0, 494.0, 496.0, 498.0, 500.0, 502.0, 504.0, 506.0, 508.0, 510.0, 512.0, 514.0, 516.0, 518.0, 520.0, 522.0, 524.0, 526.0, 528.0, 530.0, 532.0, 534.0, 536.0, 538.0, 540.0, 542.0, 544.0, 546.0, 548.0, 550.0, 552.0, 554.0, 556.0, 558.0, 560.0, 562.0, 564.0, 566.0000000000001, 568.0000000000001, 570.0000000000001, 572.0000000000001, 574.0000000000001, 576.0000000000001, 578.0, 580.0, 582.0, 584.0, 586.0, 588.0, 590.0, 592.0, 594.0, 596.0, 598.0, 600.0, 602.0, 604.0, 606.0, 608.0, 610.0, 612.0, 614.0, 616.0, 618.0, 620.0, 622.0, 624.0, 626.0, 628.0, 630.0, 632.0, 634.0, 636.0, 638.0, 640.0, 642.0, 644.0, 646.0, 648.0, 650.0, 652.0, 654.0, 656.0, 658.0, 660.0, 662.0, 664.0, 666.0, 668.0], [-0.06881431507540459, 0.09607329730283931, 0.3644776572753572, 0.7252476484810142, 1.1482358541135558, 1.5900790305922565, 1.9947718444384952, 2.3012364769355, 2.463384422043182, 2.4508784951835993, 2.249022919655184, 1.8628338497596124, 1.312907220252065, 0.6339741494596594, -0.12582284904820917, -0.9052989539873848, -1.6326465770909118, -2.2323738796094026, -2.635080631818928, -2.790206787226128, -2.678277611447163, -2.323209791519724, -1.7995081880929673, -1.2194246668214364, -0.7115347454004937, -0.39689511268482214, -0.36359798166537516, -0.6385377882106074, -1.1715347720572957, -1.849254425003667, -2.5161848900654062, -3.0066639399183286, -3.191649842725317, -3.012837964461216, -2.4986188999264805, -1.7577993970133097, -0.9532555579913904, -0.27010759688933206, 0.13471960847734366, 0.17788452218426887, -0.1360779625853512, -0.7189196545402954, -1.430314343932639, -2.117002978809945, -2.6371054771378954, -2.8879556086629985, -2.8336718491798694, -2.507890202177039, -1.9823071107030543, -1.340401189007346, -0.6647828040107671, -0.01826061928652689, 0.5606426014884942, 1.0466032617756156, 1.422296866166889, 1.6706951017011973, 1.7644299961739183, 1.6849017882743464, 1.4312203721343815, 1.0217433280668469, 0.5103311357549101, -0.01947153839484872, -0.467476689946592, -0.7370202627208926, -0.7579807769628748, -0.5001027128979383, 0.018186618862957138, 0.734642455745232, 1.5666559901251578, 2.440587775305744, 3.3063604180897004, 4.150829378760155, 5.005606328945041, 5.938588567525017, 7.038183634373722, 8.38562835632006, 10.033860465128527, 12.006298447657974, 14.301039740006672, 16.889639498879564, 19.727265768612465, 22.773691857695248, 26.00836254469079, 29.43406836897654, 33.07187303456872, 36.95866776065195, 41.1327389163273, 45.60695150486353, 50.3574692591464, 55.32432563064276, 60.415956221568585, 65.52533585167257, 70.54113520256266, 75.3713280619736, 79.97522479664671, 84.37382066964598, 88.64322300421065, 92.88762704614362, 97.21934720648193, 101.73849351451595, 106.49687463814193, 111.47914778483451, 116.61193210671735, 121.77628893215078, 126.83177924965524, 131.64785875224604, 136.11565117779438, 140.16973712098547, 143.79678606295664, 147.0264714608678, 149.91109065813066, 152.4950817781358, 154.80090869097987, 156.818639086612, 158.50160020934916, 159.76817701404065, 160.51769484906097, 160.64951068802088, 160.08978379730638, 158.81767977462897, 156.8528454974025, 154.2545964277134, 151.1280300132683, 147.5923054116302, 143.7615218768737, 139.7293069428232, 135.54980609760077, 131.24026243457152, 126.7835114278036, 122.13713094146979, 117.24989896461898, 112.0834095873991, 106.63310802212601, 100.92639885066018, 95.01700172255045, 88.9915953025477, 82.9429134481876, 76.94227247244615, 71.04870774678814, 65.2986307944837, 59.70859217846498, 54.30545864583081, 49.119870527068635, 44.186722007048076, 39.56032605303622, 35.29658796814627, 31.431825405191532, 27.966451065275507, 24.86108557259398, 22.0445538796447, 19.42149520609297, 16.885606509741415, 14.348486296232416, 11.760429229379444, 9.114207068872332, 6.448356274855893, 3.8317032466940284, 1.3488838460359132, -0.9065806351016081, -2.8405105338003915, -4.377897364708641, -5.480971431959148, -6.143520272503515, -6.390131899766828, -6.282255490864902, -5.915669361271165, -5.410456835424315, -4.903990674938763, -4.534696634619286, -4.410287020899148, -4.584763718792513, -5.049341775668862, -5.729849092034441, -6.504112631912852, -7.219857835895809, -7.7248195200007315, -7.9089933544977615, -7.728628623994307, -7.22062031154606, -6.495710091486014, -5.718620317038937, -5.072143316474815, -4.717691909478429, -4.764053926594212, -5.251450436122838, -6.14174084963954, -7.325865049555647, -8.664568954449564, -10.010116610875343, -11.227134710478508, -12.220573840138305, -12.944084749793188, -13.400069799534464, -13.631289817268335, -13.700533417075784, -13.677232272439966, -13.636956704063593, -13.647871089746193, -13.752285834472332, -13.970885495780399, -14.308330205002553, -14.743652608284703, -15.225130872746616, -15.680569271243396, -16.031396548628326, -16.1992974282664, -16.119734134243277, -15.757864924841835, -15.120105041454307, -14.248061226823198, -13.212235081252151, -12.113047784915189, -11.050736165073959, -10.108119138430823, -9.347242624426983, -8.789572970239337, -8.417899246133882, -8.186198935951003, -8.031150973029394, -7.893975014500983, -7.720085420428196, -7.473200586200749, -7.159241202679578, -6.817194970822276, -6.506770396938463, -6.293493174798042, -6.235552094648289, -6.371534015311768, -6.695650630961836, -7.152448241567073, -7.647853231922961, -8.060023644258614, -8.273673657272733, -8.223921736744964, -7.935281787565511, -7.541125661169236, -7.260531380260961, -7.353591414220748, -8.042218018859776, -9.392549480866837, -11.222711750997524, -13.060700178068526, -14.146023686893239, -13.53062614867125, -10.271379164295695, -3.649304631861405, 6.605181612743754, 20.152749704483995, 36.00505884460037, 